vi "IR Opo Main.vi"() -> ()   [LabVIEW 2016] (continued)
          }
        }
        n211 = call "uc480_SubVI_Example_MemoryAllocation.vi"(".NET (Reference)"=w417, "Error In"=w414) -> ("Bits/Pixel 2"=→"Bits/Pixel":i32, "Width"=→"Width":i32, "Serial Number"=→"Serial Number":string, "Height"=→"Height":i32, "Error Out"=w454:errorcluster)  [unwired: 13 in]
      }
      frame "Start live" {
        # "Has acquisition started?"
        # "Start Acquisition"
        n212 = property class="Camera"(reference=w518, error in=w519) -> (error out=w528:errorcluster, "Acquisition"=w527:refnum<k24>)  [unwired: 1 out]
        n213 = invoke class="Acquisition" method="HasStarted"(reference=w527, error in=w528) -> (reference out=w523:refnum<k24>, error out=w522:errorcluster, "HasStarted"=w521:i32, "bValue"=w526:bool)  [unwired: 2 in]
        n214 = control-ref of="Load Parameter"() -> (w511:refnum<vi>)
        n215 = control-ref of="Stop Live"() -> (w509:refnum<vi>)
        n216 = control-ref of="Start Live"() -> (w514:refnum<vi>)
        n217 = property class="Bool"(reference=w514, "Disabled"=u8 2 ("Deaktiviert")) -> (reference out=w503:refnum<vi>, error out=w502:errorcluster)  [unwired: 1 in]
        n218 = property class="Bool"(reference=w511, "Disabled"=u8 2 ("Deaktiviert")) -> (reference out=w505:refnum<vi>, error out=w504:errorcluster)  [unwired: 1 in]
        n219 = invoke class="Acquisition" method="ToString"(reference=w523, error in=w522) -> (error out=w525:errorcluster, "ToString"=w524:string)  [unwired: 1 in, 1 out]
        n220 = property class="Bool"(reference=w509, "Disabled"=u8 0 ("Deaktiviert")) -> (reference out=w507:refnum<vi>, error out=w506:errorcluster)  [unwired: 1 in]
        n221 = call "uc480_Error_Handling.vi"("Error Code"=w521, "Error String"=w524, "Error In"=w525) -> ("Error Out"=w520:errorcluster)  [unwired: 8 in]
        n222 = Close Reference(reference=w507, error in (no error)=w506) -> ()  [unwired: 1 out]
        n223 = Close Reference(reference=w503, error in (no error)=w502) -> ()  [unwired: 1 out]
        n224 = Close Reference(reference=w505, error in (no error)=w504) -> ()  [unwired: 1 out]
        n225 = Get Date/Time In Seconds() -> (seconds since 1Jan1904=w497:timestamp)
        n226 = Format Date/Time String(time format string (%c)="%m/%d/%y - %I:%M %p  ", seconds (now)=w497) -> (date/time string=w496:string)  [unwired: 1 in]
        n227 = Concatenate Strings(w496, "Camera started", "\r") -> (w501:string)
        n228 = invoke on="Log" class="Str" method="Append String"("string"=w501) -> (error out=w494:errorcluster)  [unwired: 3 in, 3 out]
        n229 = property on="Log" class="Str"(error in=w494, "Text.Scroll Position"=u32 500000) -> ()  [unwired: 1 in, 2 out]
        n230 = case shown="False" w526 {
          tunnel: [w531 w541] -> w515
          tunnel: w520 -> [w537 w541]
          tunnel: w518 -> [w536 w540]
          tunnel: [w536 w540] -> w517
          frame False {
            w529 = 1 items=["IS_DONT_WAIT", "IS_WAIT"] ("Wait")
            n231 = property class="Camera"(reference=w536, error in=w537) -> (error out=w538:errorcluster, "Acquisition"=w539:refnum<k24>)  [unwired: 1 out]
            n232 = invoke class="Acquisition" method="Capture"(reference=w539, error in=w538, "param"=w529) -> (reference out=w532:refnum<k24>, error out=w533:errorcluster, "Capture"=w530:i32)  [unwired: 1 in, 1 out]
            n233 = invoke class="Acquisition" method="ToString"(reference=w532, error in=w533) -> (error out=w535:errorcluster, "ToString"=w534:string)  [unwired: 1 in, 1 out]
            n234 = call "uc480_Error_Handling.vi"("Error Code"=w530, "Error String"=w534, "Error In"=w535) -> ("Error Out"=w531:errorcluster)  [unwired: 8 in]
          }
          frame True {
          }
        }
      }
    }
    n235 = call "uc480_SubVI_Example_SyncEventLoop.vi"("Error In"=w55, "use sync"=w57, ".NET (Reference)"=w56) -> ("Error Out"=w53:errorcluster, "Synchronize (ms)"=w54:dbl)  [unwired: 7 in]
    "Error Out" <- w53
    n236 = Wait Until Next ms Multiple(millisecond multiple=w54) -> ()  [unwired: 1 out]
  }
  n237 = flat-sequence "Initialization sequence" {
    tunnel: [w596] -> w20
    tunnel: w20 -> [w658]
    tunnel: [w641] -> w15
    tunnel: [w640] -> w14
    tunnel: [w639] -> w16
    tunnel: [w638] -> w13
    tunnel: [w637] -> w12
    tunnel: w16 -> [w669]
    tunnel: w15 -> [w668]
    tunnel: w14 -> [w667]
    tunnel: [w666] -> w11
    tunnel: w13 -> [w665]
    tunnel: w12 -> [w664]
    tunnel: [w661] -> w10
    tunnel: [w660] -> w6
    tunnel: w11 -> [w689]
    tunnel: [w689] -> w9
    tunnel: w10 -> [w688]
    tunnel: [w687] -> w7
    tunnel: w6 -> [w687]
    tunnel: w9 -> [w699]
    tunnel: [w699] -> w8
    tunnel: w7 -> [w698]
    tunnel: [w708] -> w17
    tunnel: w8 -> [w708]
    tunnel: [w713] -> w18
    tunnel: w17 -> [w713]
    tunnel: [w726] -> w19
    tunnel: w18 -> [w726]
    tunnel: [w728] -> w5
    tunnel: w19 -> [w728]
    tunnel: w5 -> [w732]
    tunnel: [w732] -> w4
    tunnel: w4 -> [w734]
    tunnel: [w734] -> w3
    tunnel: w3 -> [w736]
    tunnel: [w736] -> w2
    tunnel: w2 -> [w738]
    tunnel: [w738] -> w1
    tunnel: w1 -> [w739]
    frame #0 {
      w542 = FALSE ("Visible")
      # "Put name of .ini file here (i.e., opotek_27015_849_847.ini).\nThe .ini file must be in the 'c:\\opotek' directory"
      n238 = control-ref of="This VI"() -> (w570:refnum<vi>)
      n239 = invoke class="VI" method="Default Vals.Reinit All"(reference=w570) -> ()  [unwired: 2 in, 3 out]
      n240 = property on="Axes Manual Control" class="Bool (strict)"("Visible"=w542) -> ()  [unwired: 2 in, 2 out]
      n241 = property on="Home Axes" class="Bool"("Visible"=w542) -> ()  [unwired: 2 in, 2 out]
      n242 = call "File Dialog"("start path"=path "C:/opotek", "pattern (all files)"="*.ini*") -> ("selected path"=w565:path, "cancelled"=w564:bool, "error out"=w563:errorcluster)  [unwired: 10 in, 1 out]
      n243 = case shown="False" w564 {
        tunnel: w563 -> [w579 w581]
        tunnel: [w579 w580] -> w562
        frame False {
          n244 = Get Date/Time In Seconds() -> (seconds since 1Jan1904=w574:timestamp)
          n245 = Format Date/Time String(time format string (%c)="%m/%d/%y -%I:%M %p  ", seconds (now)=w574) -> (date/time string=w573:string)  [unwired: 1 in]
          n246 = Concatenate Strings(w573, "Initializing the OPO laser..." ("Initialiazation"), "\r") -> (w578:string)
          n247 = invoke on="Log" class="Str" method="Append String"("string"=w578) -> (error out=w571:errorcluster)  [unwired: 3 in, 3 out]
          n248 = property on="Log" class="Str"(error in=w571, "Text.Scroll Position"=u32 500000) -> ()  [unwired: 1 in, 2 out]
        }
        frame True {
          n249 = call <vilib>:"Clear Errors.vi"("error in (no error)"=w581) -> ("error out"=w580:errorcluster)  [unwired: 5 in, 1 out]
        }
      }
      n250 = Strip Path(path=w565) -> (name=w568:string)  [unwired: 1 out]
      n251 = dll-call lib="D:/Fabrizio/Labview Projects/IR OPO Controller/Branches/XPS version/OPOTEK.dll" fn="OPOTEK_Init"("INI_File"=w568) -> ("motorCOMPort"=w561:i32, "laserCOMPort"=w560:i32, "error_Code"=→"error_Code":i32)  [unwired: 8 in, 2 out]
      "motorCOMPort" <- w561
      "laserCOMPort" <- w560
      n252 = Number To Decimal String(number=w561) -> (decimal integer string=w559:string)  [unwired: 1 in]
      n253 = Number To Decimal String(number=w560) -> (decimal integer string=w557:string)  [unwired: 1 in]
      n254 = Concatenate Strings("Motor found on port: " ("string"), w559) -> (w555:string)
      n255 = Concatenate Strings("Laser found on port: " ("string"), w557) -> (w554:string)
      n256 = Build Array(w555) -> (w553:string[])
      n257 = Build Array(w554) -> (w552:string[])
      n258 = Build Array(w553, w552) -> (w551:string[][])
      n259 = Get Date/Time In Seconds() -> (seconds since 1Jan1904=w546:timestamp)
      n260 = Format Date/Time String(time format string (%c)="%m/%d/%y -%I:%M %p  ", seconds (now)=w546) -> (date/time string=w545:string)  [unwired: 1 in]
      n261 = Array To Spreadsheet String(array=w551, 3:"%s" ("format string")) -> (spreadsheet string=w548:string)  [unwired: 1 in]
      n262 = Concatenate Strings(w545, w548) -> (w549:string)
      n263 = invoke on="Log" class="Str" method="Append String"("string"=w549) -> (error out=w543:errorcluster)  [unwired: 3 in, 3 out]
      n264 = property on="Log" class="Str"(error in=w543, "Text.Scroll Position"=u32 500000) -> ()  [unwired: 1 in, 2 out]
      n265 = call <vilib>:"Simple Error Handler.vi"("error in (no error)"=w562) -> ()  [unwired: 4 in, 5 out]
    }
    frame #1 {
      w614 = "ROI Processing" ("section")
      w622 = "XPS" ("section")
      n266 = control-ref of="This VI"() -> (w636:refnum<vi>)
      n267 = property class="VI"(reference=w636) -> ("Path"=w634:path)  [unwired: 1 in, 2 out]
      n268 = Strip Path(path=w634) -> (stripped path=w633:path)  [unwired: 1 out]
      n269 = Build Path(base path=w633, name or relative path="General_Configuration.ini") -> (appended path=w624:path)
      n270 = call <vilib>:"Open Config Data.vi"("create file if necessary (T)"=FALSE, "configuration file path"=w624) -> ("error out"=w623:errorcluster, "refnum"=w595:T6)  [unwired: 7 in, 1 out]
      n271 = call-poly <vilib>:"Read Key.vi"("section"="Communication", "default value"="192.168.254.254", "key"="XPSPort", "refnum"=w595) -> ("error out"=w589:errorcluster, "value"=→"XPS_Address":string)  [unwired: 4 in, 2 out]
      n272 = call-poly <vilib>:"Read Key.vi"("section"=w622, "error in (no error)"=w623, "default value"=1.0, "key"="InitialVelocity", "refnum"=w595) -> ("error out"=w588:errorcluster, "value"=→"Velocity":dbl)  [unwired: 3 in, 2 out]
      n273 = call-poly <vilib>:"Read Key.vi"("section"=w622, "default value"=20.0, "key"="Acceleration", "refnum"=w595) -> ("error out"=w587:errorcluster, "value"=→"Acceleration":dbl)  [unwired: 4 in, 2 out]
      n274 = call-poly <vilib>:"Read Key.vi"("section"="Laser" ("key"), "default value"=0, "key"="Wavelenght", "refnum"=w595) -> ("error out"=w586:errorcluster, "value"=→"Default Wavelenght":i32)  [unwired: 4 in, 2 out]
      n275 = Merge Errors(w589, w588, w587, w586) -> (w590:errorcluster)
      n276 = call-poly <vilib>:"Read Key.vi"("section"=w614, "key"="Pixel Size", "refnum"=w595) -> ("error out"=w605:errorcluster, "value"=w594:dbl)  [unwired: 5 in, 2 out]
      n277 = call-poly <vilib>:"Read Key.vi"("section"=w614, "key"="Heigth step divider", "refnum"=w595) -> ("error out"=w604:errorcluster, "value"=w593:i32)  [unwired: 5 in, 2 out]
      n278 = call-poly <vilib>:"Read Key.vi"("section"=w614, "key"="Precision (%)", "refnum"=w595) -> ("error out"=w603:errorcluster, "value"=w591:dbl)  [unwired: 5 in, 2 out]
      n279 = call-poly <vilib>:"Read Key.vi"("section"=w614, "key"="Sampling speed", "refnum"=w595) -> ("error out"=w602:errorcluster, "value"=w592:i32)  [unwired: 5 in, 2 out]
      n280 = call-poly <vilib>:"Read Key.vi"("section"=w614, "key"="Width", "refnum"=w595) -> ("error out"=w601:errorcluster, "value"=w585:i32)  [unwired: 5 in, 2 out]
      n281 = call-poly <vilib>:"Read Key.vi"("section"=w614, "key"="Height", "refnum"=w595) -> ("error out"=w600:errorcluster, "value"=w584:i32)  [unwired: 5 in, 2 out]
      n282 = call-poly <vilib>:"Read Key.vi"("section"=w614, "key"="X offset", "refnum"=w595) -> ("error out"=w599:errorcluster, "value"=w583:i32)  [unwired: 5 in, 2 out]
      n283 = call-poly <vilib>:"Read Key.vi"("section"=w614, "key"="Y offset", "refnum"=w595) -> ("error out"=w598:errorcluster, "value"=w582:i32)  [unwired: 5 in, 2 out]
      n284 = Merge Errors(w605, w604, w603, w602, w601, w600, w599, w598, w590) -> (w597:errorcluster)
      n285 = local write "Height  step \ndivider"(w593) -> ()
      n286 = call <vilib>:"Close Config Data.vi"("error in (no error)"=w597, "refnum"=w595) -> ("error out"=w596:errorcluster)  [unwired: 8 in, 1 out]
      n287 = local write "Speed (µm/s)"(w592) -> ()
      n288 = local write "Precision (%)"(w591) -> ()
      n289 = local write "Pixel size"(w594) -> ()
      n290 = local write "Heigth (µm)"(w584) -> ()
      n291 = local write "Width (µm)"(w585) -> ()
      n292 = local write "Y offset"(w582) -> ()
      n293 = local write "X offset"(w583) -> ()
    }
    frame #2 {
      w642 = "\r"
      n294 = local read "XPS_Address"() -> (w659:string)
      n295 = call <userlib>:"Open TCP-IP.vi"("error in (no error)"=w658, "IP address"=w659) -> ("error out"=w656:errorcluster, "Connection ID"=w657:T7)  [unwired: 4 in, 4 out]
      n296 = call <userlib>:"Objects List Get.vi"("error in (no error)"=w656, "connection ID in"=w657) -> ("error out"=w637:errorcluster, "XPS error out"=w638:errorcluster, "connection ID out"=w639:T7, "Groups"=w655:string[])  [unwired: 4 in, 2 out]
      n297 = Get Date/Time In Seconds() -> (seconds since 1Jan1904=w651:timestamp)
      n298 = Format Date/Time String(time format string (%c)="%m/%d/%y -%I:%M %p  ", seconds (now)=w651) -> (date/time string=w644:string)  [unwired: 1 in]
      n299 = Index Array(array=w655) -> (element=w640:string)  [unwired: 1 in]
      "Axis 1" <- w640
      n300 = Index Array(array=w655, index=1) -> (element=w641:string)
      "Axis 2" <- w641
      n301 = Concatenate Strings(w644, "Axis 1: " ("Initialiazation"), w640, w642) -> (w653:string)
      n302 = Concatenate Strings(w644, "Axis 2: " ("Initialiazation"), w641, w642) -> (w645:string)
      n303 = invoke on="Log" class="Str" method="Append String"("string"=w653) -> (error out=w649:errorcluster)  [unwired: 3 in, 3 out]
      n304 = invoke on="Log" class="Str" method="Append String"("string"=w645) -> (error out=w646:errorcluster)  [unwired: 3 in, 3 out]
      n305 = property on="Log" class="Str"(error in=w649, "Text.Scroll Position"=u32 500000) -> ()  [unwired: 1 in, 2 out]
      n306 = property on="Log" class="Str"(error in=w646, "Text.Scroll Position"=u32 500000) -> ()  [unwired: 1 in, 2 out]
    }
    frame #3 {
      w683 = "Ready"
      n307 = call "Get Stages Status.vi"("error in (no error)"=w664, "XPS error in (no error)"=w665, "Group Name (250 c max)"=w667, "connection ID in"=w669) -> ("error out"=w674:errorcluster, "XPS error out"=w675:errorcluster, "Group Status String"=w671:string, "connection ID out"=w676:T7)  [unwired: 3 in, 1 out]
      n308 = call "Get Stages Status.vi"("error in (no error)"=w674, "XPS error in (no error)"=w675, "Group Name (250 c max)"=w668, "connection ID in"=w676) -> ("error out"=w672:errorcluster, "XPS error out"=w662:errorcluster, "Group Status String"=w670:string, "connection ID out"=w673:T7)  [unwired: 3 in, 1 out]
      n309 = String Subset(string=w671, offset (0)=0, length (rest)=5 ("length (rest)")) -> (substring=w681:string)
      n310 = Bundle(cluster="Axis Initial Parameters", "Velocity (units/seconds)"=5.0) -> (w685:T1)  [unwired: 3 in]
      n311 = call <userlib>:"Close TCP-IP.vi"("error in (no error)"=w672, "connection ID in"=w673) -> ("Error out"=w663:errorcluster)  [unwired: 9 in]
      n312 = local write "Axis Initial Parameters"(w685) -> ()
      n313 = String Subset(string=w670, offset (0)=0, length (rest)=5 ("length (rest)")) -> (substring=w682:string)
      n314 = call <vilib>:"Simple Error Handler.vi"("error in (no error)"=w663) -> ()  [unwired: 4 in, 5 out]
      n315 = call <vilib>:"Simple Error Handler.vi"("error in (no error)"=w662) -> ()  [unwired: 4 in, 5 out]
      n316 = Equal?(x=w681, y=w683) -> (x = y?=w661:bool)
      n317 = Equal?(x=w683, y=w682) -> (x = y?=w660:bool)
      n318 = And(x=w661, y=w660) -> (x .and. y?=w666:bool)
    }
    frame #4 {
      n319 = case shown="True" w688 {
        frame False {
        }
        frame True {
          (unwired) u32 500000 ("Text.Scroll Position")
          n320 = Get Date/Time In Seconds() -> (seconds since 1Jan1904=w694:timestamp)
          n321 = Format Date/Time String(time format string (%c)="%m/%d/%y -%I:%M %p  ", seconds (now)=w694) -> (date/time string=w693:string)  [unwired: 1 in]
          n322 = Concatenate Strings(w693, "Axis 1 ready" ("Initialiazation"), "\r") -> (w691:string)
          n323 = invoke on="Log" class="Str" method="Append String"("string"=w691) -> (error out=w692:errorcluster)  [unwired: 3 in, 3 out]
          n324 = property on="Log" class="Str"(error in=w692, "Text.Scroll Position"=u32 500000) -> ()  [unwired: 1 in, 2 out]
        }
      }
    }
    frame #5 {
      n325 = case shown="True" w698 {
        frame False {
        }
        frame True {
          (unwired) u32 500000 ("Text.Scroll Position")
          n326 = Get Date/Time In Seconds() -> (seconds since 1Jan1904=w704:timestamp)
          n327 = Format Date/Time String(time format string (%c)="%m/%d/%y -%I:%M %p  ", seconds (now)=w704) -> (date/time string=w703:string)  [unwired: 1 in]
          n328 = Concatenate Strings(w703, "Axis 2 ready" ("Initialiazation"), "\r") -> (w701:string)
          n329 = invoke on="Log" class="Str" method="Append String"("string"=w701) -> (error out=w702:errorcluster)  [unwired: 3 in, 3 out]
          n330 = property on="Log" class="Str"(error in=w702, "Text.Scroll Position"=u32 500000) -> ()  [unwired: 1 in, 2 out]
        }
      }
    }
    frame #6 {
      n331 = dll-call lib="D:/Fabrizio/Labview Projects/IR OPO Controller/Branches/XPS version/OPOTEK.dll" fn="OPOTEK_SelectConfiguration"("configuration"=u8 1 ("configuration 2")) -> ("wavelength_Low"=→"Min":dbl, "wavelength_High"=→"Max":dbl, "error_Code"=→"error_Code 2":i32)  [unwired: 8 in, 2 out]
    }
    frame #7 {
      w723 = FALSE ("Visible")
      w719 = u8 1 ("Response to Value Outside Limits:Maximum")
      # "Set defaults"
      n332 = local write "Flash lamp - Q Switch delay (%)"(i16 0 ("Energy")) -> ()
      n333 = local write "Alignment \ndiode"(TRUE ("Alignment diode")) -> ()
      n334 = local write "Repetition \nRate"(enum16{"1", "2", "5", "10", "20"}."20" ("Rep. Rate Divider")) -> ()
      n335 = local read "Max"() -> (w716:dbl)
      n336 = local read "Min"() -> (w717:dbl)
      n337 = call "IR_Alignment_Diode.vi"("AD Action"=enum16{"AD Off", "AD On"}."AD On") -> ()  [unwired: 14 in, 1 out]
      n338 = property on="LAMP" class="Bool (strict)"("BoolText.Text"="LAMP OFF" ("Boolean Text.Text")) -> ()  [unwired: 2 in, 2 out]
      n339 = property on="Laser Operation" class="Bool (strict)"("Blinking"=w723) -> ()  [unwired: 2 in, 2 out]
      n340 = property on="Capture" class="Bool"("Visible"=w723) -> ()  [unwired: 2 in, 2 out]
      n341 = property on="LASER" class="Bool (strict)"("BoolText.Text"="LASER OFF" ("Boolean Text.Text"), "Visible"=FALSE) -> ()  [unwired: 2 in, 2 out]
      n342 = property on="Wavelength" class="DigNum (strict)"("Increment"=1.0 ("Data Entry Limits:Increment"), "Maximum"=w716, "Minimum"=w717, "OutOfRngActMax"=w719, "OutOfRngActMin"=w719) -> ()  [unwired: 2 in, 2 out]
    }
    frame #8 {
      n343 = local read "Default Wavelenght"() -> (w727:i32)
      n344 = local write "Wavelength"(w727) -> ()
      n345 = call "IR_Wavelength_Tuning.vi"("Wavelength (nm)"=w727) -> ()  [unwired: 14 in, 1 out]
    }
    frame #9 {
      w729 = i16 100 ("Energy (0 - 100)")
      n346 = call "IR_Laser_Control.vi"("Action"=T5."Adjust Energy", "Energy (0 - 100)"=w729) -> ()  [unwired: 13 in, 1 out]
      n347 = local write "Flash lamp - Q Switch delay (%)"(w729) -> ()
    }
    frame #10 {
      n348 = local write "Camera Status"("Init camera" ("Camera Status")) -> ()
    }
    frame #11 {
      n349 = Wait (ms)(milliseconds to wait=u32 1000) -> ()  [unwired: 1 out]
    }
    frame #12 {
      n350 = local write "Camera Status"("Start live") -> ()
    }
    frame #13 {
      n351 = Wait (ms)(milliseconds to wait=u32 1000) -> ()  [unwired: 1 out]
    }
    frame #14 {
      n352 = case shown="True" w739 {
        frame False {
          n353 = One Button Dialog(message="Axes not ready") -> ()  [unwired: 1 in, 1 out]
        }
        frame True {
          n354 = Get Date/Time In Seconds() -> (seconds since 1Jan1904=w746:timestamp)
          n355 = property on="Home Axes" class="Bool"("Visible"=TRUE) -> ()  [unwired: 2 in, 2 out]
          n356 = property on="Axes Manual Control" class="Bool (strict)"("Visible"=TRUE) -> ()  [unwired: 2 in, 2 out]
          n357 = Format Date/Time String(time format string (%c)="%m/%d/%y -%I:%M %p  ", seconds (now)=w746) -> (date/time string=w747:string)  [unwired: 1 in]
          n358 = Concatenate Strings(w747, "System ready" ("Initialiazation"), "\r") -> (w749:string)
          n359 = invoke on="Log" class="Str" method="Append String"("string"=w749) -> (error out=w748:errorcluster)  [unwired: 3 in, 3 out]
          n360 = property on="Log" class="Str"(error in=w748, "Text.Scroll Position"=u32 500000) -> ()  [unwired: 1 in, 2 out]
        }
      }
    }
  }
  n361 = while "Laser control & Stages Control" {
    stop <- w761 stop-if-true
    n362 = local read "XPS_Address"() -> (w753:string)
    n363 = local read "Axis 2"() -> (w751:string)
    n364 = local read "Axis 1"() -> (w752:string)
    n365 = event shown="[12] \"Process Image\": Value Change" {
      selector: _ -> [_ _ _ _ _ _ _ _ _ _ _ _ _ _ _ _ _]
      dyn-events: _ -> [_ _ _ _ _ _ _ _ _ _ _ _ _ _ _ _ _]
      timeout: _ -> [_ _ _ _ _ _ _ _ _ _ _ _ _ _ _ _ _]
      tunnel: [_ _ _ _ _ w832 _ _ _ _ _ _ _ _ _ _ _] -> w761
      tunnel: [w765 w772 w791 w814 w821 _ _ _ _ w887 w914 _ w989 "" ("StringOut") w1183 _ w1307] -> w754
      tunnel: w753 -> [_ _ _ _ _ _ _ _ _ _ w917 _ _ w1102 w1182 _ w1294]
      tunnel: w752 -> [_ _ _ _ _ _ _ _ _ _ w916 _ _ w1101 w1181 _ w1293]
      tunnel: w751 -> [_ _ _ _ _ _ _ _ _ _ w915 _ _ w1100 w1180 _ w1292]
      event "Flash lamp - Q Switch delay (%)": Value Change {
        n366 = event-data() -> ()  [unwired: 1 in, 6 out]
        n367 = local read "Flash lamp - Q Switch delay (%)"() -> (w769:i16)
        n368 = call "IR_Laser_Control.vi"("Action"=T5."Adjust Energy", "Energy (0 - 100)"=w769) -> ()  [unwired: 13 in, 1 out]
        n369 = Number To Decimal String(number=w769, width (-)=i16 3) -> (decimal integer string=w767:string)
        n370 = Concatenate Strings("Energy set to: " ("string"), w767) -> (w765:string)
      }
      event "LAMP": Value Change {
        n371 = event-data() -> ()  [unwired: 1 in, 6 out]
        n372 = case shown="True" "LAMP" {
          tunnel: ["Lamp has been switched off" w777] -> w772
          frame False {
            w774 = FALSE ("Visible")
            n373 = property on="LASER" class="Bool (strict)"("Visible"=w774) -> ()  [unwired: 2 in, 2 out]
            n374 = property on="Capture" class="Bool"("Visible"=w774) -> ()  [unwired: 2 in, 2 out]
            n375 = call "IR_Laser_Control.vi"("Action"=T5."Lamp OFF") -> ()  [unwired: 14 in, 1 out]
            n376 = property on="LAMP" class="Bool (strict)"("BoolText.Text"="LAMP OFF" ("Boolean Text.Text")) -> ()  [unwired: 2 in, 2 out]
          }
          frame True {
            n377 = flat-sequence {
              tunnel: ["Lamp has been switched on"] -> w777
              frame #0 {
                n378 = while {
                  i -> [w782]
                  stop <- w785 stop-if-true
                  n379 = Wait Until Next ms Multiple(millisecond multiple=u32 1000) -> ()  [unwired: 1 out]
                  n380 = Equal?(x=10, y=w782) -> (x = y?=w785:bool)
                  n381 = Subtract(x=10, y=w782) -> (x-y=w780:i32)
                  n382 = Number To Decimal String(number=w780) -> (decimal integer string=w781:string)  [unwired: 1 in]
                  n383 = property on="LAMP" class="Bool (strict)"("BoolText.Text"=w781) -> ()  [unwired: 2 in, 2 out]
                }
                n384 = Wait (ms)(milliseconds to wait=u32 10000) -> ()  [unwired: 1 out]
                n385 = call "IR_Laser_Control.vi"("Action"=T5."Lamp ON") -> ()  [unwired: 14 in, 1 out]
              }
              frame #1 {
                w788 = TRUE ("Visible")
                n386 = property on="LASER" class="Bool (strict)"("Visible"=w788) -> ()  [unwired: 2 in, 2 out]
                n387 = property on="Capture" class="Bool"("Visible"=w788) -> ()  [unwired: 2 in, 2 out]
                n388 = property on="LAMP" class="Bool (strict)"("BoolText.Text"="LAMP ON" ("Boolean Text.Text")) -> ()  [unwired: 2 in, 2 out]
              }
            }
          }
        }
      }
      event "LASER": Value Change {
        n389 = event-data() -> ()  [unwired: 1 in, 6 out]
        n390 = case shown="True" "LASER" {
          tunnel: [w796 w802] -> w792
          tunnel: ["Q-Switch has switched off" w801] -> w791
          frame False {
            w796 = FALSE ("Boolean")
            n391 = local read "Alignment \ndiode"() -> (w793:bool)
            n392 = property on="Capture" class="Bool"("Visible"=TRUE) -> ()  [unwired: 2 in, 2 out]
            n393 = case shown="False" w793 {
              frame False {
                n394 = call "IR_Alignment_Diode.vi"("AD Action"=enum16{"AD Off", "AD On"}."AD Off") -> ()  [unwired: 14 in, 1 out]
              }
              frame True {
                n395 = call "IR_Alignment_Diode.vi"("AD Action"=enum16{"AD Off", "AD On"}."AD On") -> ()  [unwired: 14 in, 1 out]
              }
            }
            n396 = call "IR_Laser_Control.vi"("Action"=T5."Q-switch OFF") -> ()  [unwired: 14 in, 1 out]
            n397 = property on="LASER" class="Bool (strict)"("BoolText.Text"="LASER OFF" ("Boolean Text.Text"), "Value"=w796) -> ()  [unwired: 2 in, 2 out]
            n398 = property on="Laser Operation" class="Bool (strict)"("Blinking"=w796) -> ()  [unwired: 2 in, 2 out]
          }
          frame True {
            n399 = property on="LAMP" class="Bool (strict)"() -> ("BoolText.Text"=w805:string)  [unwired: 2 in, 2 out]
            n400 = Equal?(x=w805, y="LAMP ON") -> (x = y?=w803:bool)
            n401 = case shown="True" w803 {
              tunnel: [FALSE ("Boolean") w811] -> w802
              tunnel: ["Q-Switch has switched off" "Q-Switch has switched on"] -> w801
              frame False {
              }
              frame True {
                w811 = TRUE ("Boolean")
                n402 = property on="Capture" class="Bool"("Visible"=FALSE) -> ()  [unwired: 2 in, 2 out]
                n403 = property on="LASER" class="Bool (strict)"("BoolText.Text"="LASER ON" ("Boolean Text.Text")) -> ()  [unwired: 2 in, 2 out]
                n404 = call "IR_Alignment_Diode.vi"("AD Action"=enum16{"AD Off", "AD On"}."AD Off") -> ()  [unwired: 14 in, 1 out]
                n405 = property on="Laser Operation" class="Bool (strict)"("Blinking"=w811) -> ()  [unwired: 2 in, 2 out]
                n406 = call "IR_Laser_Control.vi"("Action"=T5."Q-switch ON") -> ()  [unwired: 14 in, 1 out]
              }
            }
          }
        }
        "Laser Operation" <- w792
      }
      event "Repetition \nRate": Value Change {
        n407 = event-data() -> ()  [unwired: 1 in, 6 out]
        n408 = local read "Repetition \nRate"() -> (w815:enum16{"1", "2", "5", "10", "20"})
        n409 = call "IR_Laser_Control.vi"("Action"=T5."Change Rep. Rate", "Rep. Rate Divider"=w815) -> ()  [unwired: 13 in, 1 out]
        n410 = Number To Decimal String(number=w815, width (-)=i16 3) -> (decimal integer string=w817:string)
        n411 = Concatenate Strings("Repetition rate set to: " ("string"), w817) -> (w814:string)
      }
      event "Tune": Value Change {
        n412 = event-data() -> ()  [unwired: 1 in, 6 out]
        n413 = case shown="True" "Tune" {
          tunnel: [_ w822] -> w821
          frame False {
          }
          frame True {
            n414 = property on="LASER" class="Bool (strict)"() -> ("BoolText.Text"=w829:string)  [unwired: 2 in, 2 out]
            n415 = Equal?(x=w829, y="LASER ON") -> (x = y?=w827:bool)
            n416 = case shown="False" w827 {
              tunnel: [w830 w831] -> w823
              frame False {
                n417 = local read "Wavelength"() -> (w830:dbl)
                n418 = call "IR_Wavelength_Tuning.vi"("Wavelength (nm)"=w830) -> ()  [unwired: 14 in, 1 out]
              }
              frame True {
                n419 = local read "Wavelength"() -> (w831:dbl)
              }
            }
            n420 = Number To Decimal String(number=w823, width (-)=i16 3) -> (decimal integer string=w825:string)
            n421 = Concatenate Strings("Wavelength set to: " ("string"), w825) -> (w822:string)
          }
        }
      }
      event "EXIT": Value Change {
        n422 = event-data() -> ()  [unwired: 1 in, 6 out]
        n423 = flat-sequence {
          tunnel: ["EXIT"] -> w832
          frame #0 {
            n424 = call "IR_Laser_Control.vi"("Action"=T5."Lamp OFF") -> ()  [unwired: 14 in, 1 out]
          }
          frame #1 {
            n425 = Wait (ms)(milliseconds to wait=u32 1000) -> ()  [unwired: 1 out]
          }
          frame #2 {
            n426 = dll-call lib="D:/Fabrizio/Labview Projects/IR OPO Controller/Branches/XPS version/OPOTEK.dll" fn="OPOTEK_Close"() -> ("error_Code"=→"error_Code 3":i32)  [unwired: 5 in, 2 out]
          }
          frame #3 {
            n427 = Wait (ms)(milliseconds to wait=u32 1000) -> ()  [unwired: 1 out]
          }
          frame #4 {
            n428 = local write "Camera Status"("Exit camera") -> ()
          }
          frame #5 {
            n429 = Wait (ms)(milliseconds to wait=u32 1000) -> ()  [unwired: 1 out]
          }
          frame #6 {
            n430 = control-ref of="This VI"() -> (w842:refnum<vi>)
            n431 = property class="VI"(reference=w842) -> ("Path"=w843:path)  [unwired: 1 in, 2 out]
            n432 = control-ref of="This Application"() -> (w858:refnum<vi>)
            n433 = Strip Path(path=w843) -> (stripped path=w852:path)  [unwired: 1 out]
            n434 = property class="App"(reference=w858) -> ("App.Kind"=w857:T10)  [unwired: 1 in, 2 out]
            n435 = Build Path(base path=w852, name or relative path="Logs") -> (appended path=w850:path)
            n436 = case shown="\"Run Time System\"" w857 {
              frame "Development System", Default {
              }
              frame "Run Time System" {
                n437 = control-ref of="This VI"() -> (w867:refnum<vi>)
                n438 = invoke class="VI" method="FP.Close"(reference=w867) -> ()  [unwired: 2 in, 3 out]
                n439 = Quit LabVIEW() -> ()  [unwired: 1 in]
              }
            }
            n440 = call <vilib>:"Check if File or Folder Exists.vi"("path"=w850) -> ("file or folder exists?"=w851:bool, "dup path"=w853:path)  [unwired: 8 in, 1 out]
            n441 = case shown="True" w851 {
              tunnel: w853 -> [w860 w861]
              tunnel: [w859 w861] -> w856
              frame False {
                n442 = Create Folder(path (use dialog)=w860) -> (created path=w859:path)  [unwired: 2 in, 2 out]
              }
              frame True {
              }
            }
            n443 = Get Date/Time In Seconds() -> (seconds since 1Jan1904=w847:timestamp)
            n444 = Format Date/Time String(time format string (%c)="%d%m%y %I-%M %p ", seconds (now)=w847) -> (date/time string=w845:string)  [unwired: 1 in]
            n445 = Concatenate Strings(w845, "Log File.txt") -> (w855:string)
            n446 = Build Path(base path=w856, name or relative path=w855) -> (appended path=w854:path)
            n447 = Open/Create/Replace File(file path (use dialog)=w854, operation (0:open)=T8."replace or create") -> (refnum out=w841:refnum<file>, cancelled=w839:bool, error out=w840:errorcluster)  [unwired: 4 in]
            n448 = case shown="False" w839 {
              tunnel: w841 -> [w866 _]
              tunnel: w840 -> [w864 _]
              frame False {
                n449 = local read "Log"() -> (w865:string)
                n450 = Write to Text File(file (use dialog)=w866, text=w865, error in=w864) -> (refnum out=w863:refnum<file>, error out=w862:errorcluster)  [unwired: 2 out]
                n451 = Close File(refnum=w863, error in=w862) -> ()  [unwired: 2 out]
              }
              frame True {
              }
            }
          }
          frame #7 {
          }
        }
      }
      event "Processing time unit", "Processi time (sec)": Value Change {
        n452 = event-data() -> ()  [unwired: 1 in, 6 out]
        n453 = local read "Processing time unit"() -> (w871:string)
        n454 = Equal?(x=w871, y="min") -> (x = y?=w869:bool)
        n455 = case shown="False" w869 {
          frame False {
            n456 = local read "Processi time (sec)"() -> (w872:i32)
            n457 = local write "Process time"(w872) -> ()
          }
          frame True {
            n458 = local read "Processi time (sec)"() -> (w874:i32)
            n459 = Quotient & Remainder(x=w874, y=60) -> (floor(x/y)=w873:i32)  [unwired: 1 out]
            n460 = local write "Process time"(w873) -> ()
          }
        }
      }
      event "Overlay MSI Image": Value Change {
        n461 = event-data() -> ()  [unwired: 1 in, 6 out]
        n462 = case shown="True" "Overlay MSI Image" {
          frame False {
          }
          frame True {
            n463 = vi-ref "MSI_Image_overlap.vi"() -> (w882:refnum<vi>)
            n464 = invoke class="VI" method="FP.Open"(reference=w882, "Activate"=TRUE ("Activate?"), "State"=T9."Standard") -> (reference out=w879:refnum<vi>)  [unwired: 2 in, 4 out]
            n465 = invoke class="VI" method="Run VI"(reference=w879, "Wait until done"=FALSE ("Wait Until Done"), "Auto Dispose Ref"=TRUE ("Auto Dispose Reference")) -> ()  [unwired: 2 in, 5 out]
          }
        }
      }
      event "Alignment \ndiode": Value Change {
        n466 = event-data() -> ()  [unwired: 1 in, 6 out]
        n467 = case shown="False" "Alignment \ndiode" {
          frame False {
            n468 = call "IR_Alignment_Diode.vi"("AD Action"=enum16{"AD Off", "AD On"}."AD Off") -> ()  [unwired: 14 in, 1 out]
          }
          frame True {
            n469 = call "IR_Alignment_Diode.vi"("AD Action"=enum16{"AD Off", "AD On"}."AD On") -> ()  [unwired: 14 in, 1 out]
          }
        }
      }
      event "Open \nManual": Value Change {
        n470 = event-data() -> ()  [unwired: 1 in, 6 out]
        n471 = case shown="True" "Open \nManual" {
          tunnel: [_ "Opening Manual" ("StringOut")] -> w887
          frame False {
          }
          frame True {
            w896 = FALSE  # wait until completion? (T)
            n472 = control-ref of="This VI"() -> (w900:refnum<vi>)
            n473 = property class="VI"(reference=w900) -> ("Path"=w899:path)  [unwired: 1 in, 2 out]
            n474 = Strip Path(path=w899) -> (stripped path=w898:path)  [unwired: 1 out]
            n475 = Build Path(base path=w898, name or relative path="LAST_Software_Manual.PDF") -> (appended path=w890:path)
            n476 = Path To String(path=w890) -> (string=w893:string)
            n477 = Concatenate Strings("cmd  /c \"", w893, "\"" ("string")) -> (w888:string)
            n478 = call <vilib>:"System Exec.vi"("run minimized? (F)"=TRUE, "wait until completion? (T)"=w896, "error in (no error)"="error in (no error)", "command line"=w888) -> ("error out"=→"error out":errorcluster)  [unwired: 4 in, 3 out]
          }
        }
      }
      event "Stages status": Value Change {
        w908 = "Ready"
        n479 = event-data() -> ()  [unwired: 1 in, 6 out]
        n480 = case shown="True" "Stages status" {
          tunnel: w917 -> [_ w930]
          tunnel: w916 -> [_ w929]
          tunnel: w915 -> [_ w928]
          tunnel: [w921 w927] -> w914
          tunnel: [w921 w925] -> w904
          tunnel: [w921 w926] -> w903
          frame False {
            w921 = ""
          }
          frame True {
            n481 = call <userlib>:"Open TCP-IP.vi"("IP address"=w930) -> ("error out"=w924:errorcluster, "Connection ID"=w931:T7)  [unwired: 8 in, 1 out]
            n482 = call <vilib>:"Simple Error Handler.vi"("error in (no error)"=w924) -> ("error?"=w922:bool, "error out"=w923:errorcluster)  [unwired: 4 in, 3 out]
            n483 = case shown="True" w922 {
              tunnel: w931 -> [w952 _]
              tunnel: w923 -> [w951 _]
              tunnel: w929 -> [w944 _]
              tunnel: w928 -> [w943 _]
              tunnel: [w942 w953] -> w927
              tunnel: [w939 w953] -> w926
              tunnel: [w935 w953] -> w925
              frame False {
                n484 = call "Get Stages Status.vi"("error in (no error)"=w951, "Group Name (250 c max)"=w944, "connection ID in"=w952) -> ("error out"=w948:errorcluster, "XPS error out"=w947:errorcluster, "Group Status String"=w939:string, "connection ID out"=w950:T7)  [unwired: 4 in, 1 out]
                n485 = call "Get Stages Status.vi"("error in (no error)"=w948, "XPS error in (no error)"=w947, "Group Name (250 c max)"=w943, "connection ID in"=w950) -> ("error out"=w945:errorcluster, "XPS error out"=w941:errorcluster, "Group Status String"=w935:string, "connection ID out"=w946:T7)  [unwired: 3 in, 1 out]
                n486 = call <vilib>:"Simple Error Handler.vi"("error source (\" \")"="Stage status" ("error source (\" \")"), "error in (no error)"=w941) -> ()  [unwired: 3 in, 5 out]
                n487 = Concatenate Strings("Axis 1 " ("string"), w939) -> (w938:string)
                n488 = call <userlib>:"Close TCP-IP.vi"("error in (no error)"=w945, "connection ID in"=w946) -> ("Error out"=w940:errorcluster)  [unwired: 9 in]
                n489 = call <vilib>:"Simple Error Handler.vi"("error source (\" \")"="TCP close Stage status" ("error source (\" \")"), "error in (no error)"=w940) -> ()  [unwired: 3 in, 5 out]
                n490 = Concatenate Strings("Axis 2 " ("string"), w935) -> (w936:string)
                n491 = Concatenate Strings(w938, " - " ("string"), w936) -> (w942:string)
              }
              frame True {
                w953 = ""
              }
            }
          }
        }
        n492 = String Subset(string=w903, offset (0)=0, length (rest)=5 ("length (rest)")) -> (substring=w907:string)
        n493 = String Subset(string=w904, offset (0)=0, length (rest)=5 ("length (rest)")) -> (substring=w909:string)
        n494 = Equal?(x=w908, y=w907) -> (x = y?=w905:bool)
        n495 = Equal?(x=w909, y=w908) -> (x = y?=w906:bool)
        n496 = And(x=w906, y=w905) -> (x .and. y?=w902:bool)
        n497 = case shown="True" w902 {
          frame False {
          }
          frame True {
            n498 = property on="Axes Manual Control" class="Bool (strict)"("Visible"=TRUE) -> ()  [unwired: 2 in, 2 out]
            n499 = property on="Home Axes" class="Bool"("Visible"=TRUE) -> ()  [unwired: 2 in, 2 out]
          }
        }
      }
      event "Save configuration": Value Change {
        n500 = event-data() -> ()  [unwired: 1 in, 6 out]
        n501 = case shown="True" "Save configuration" {
          frame False {
          }
          frame True {
            w981 = "ROI Processing" ("section")
            n502 = control-ref of="This VI"() -> (w987:refnum<vi>)
            n503 = property class="VI"(reference=w987) -> ("Path"=w986:path)  [unwired: 1 in, 2 out]
            n504 = Strip Path(path=w986) -> (stripped path=w985:path)  [unwired: 1 out]
            n505 = Build Path(base path=w985, name or relative path="General_Configuration.ini") -> (appended path=w983:path)
            n506 = local read "Heigth (µm)"() -> (w967:i32)
            n507 = local read "Width (µm)"() -> (w968:i32)
            n508 = local read "Pixel size"() -> (w979:dbl)
            n509 = local read "X offset"() -> (w966:i32)
            n510 = local read "Y offset"() -> (w965:i32)
            n511 = local read "Height  step \ndivider"() -> (w978:i32)
            n512 = call <vilib>:"Open Config Data.vi"("create file if necessary (T)"=FALSE, "configuration file path"=w983) -> ("refnum"=w955:T6)  [unwired: 7 in, 2 out]
            n513 = local read "Speed (µm/s)"() -> (w969:i32)
            n514 = local read "Precision (%)"() -> (w970:dbl)
            n515 = call-poly <vilib>:"Write Key.vi"("section"=w981, "value"=w979, "key"="Pixel Size", "refnum"=w955) -> ("error out"=w964:errorcluster)  [unwired: 5 in, 2 out]
            n516 = call-poly <vilib>:"Write Key.vi"("section"=w981, "value"=w978, "key"="Heigth step divider", "refnum"=w955) -> ("error out"=w963:errorcluster)  [unwired: 5 in, 2 out]
            n517 = call-poly <vilib>:"Write Key.vi"("section"=w981, "value"=w970, "key"="Precision (%)", "refnum"=w955) -> ("error out"=w962:errorcluster)  [unwired: 5 in, 2 out]
            n518 = call-poly <vilib>:"Write Key.vi"("section"=w981, "value"=w969, "key"="Sampling speed", "refnum"=w955) -> ("error out"=w961:errorcluster)  [unwired: 5 in, 2 out]
            n519 = call-poly <vilib>:"Write Key.vi"("section"=w981, "value"=w968, "key"="Width", "refnum"=w955) -> ("error out"=w960:errorcluster)  [unwired: 5 in, 2 out]
            n520 = call-poly <vilib>:"Write Key.vi"("section"=w981, "value"=w967, "key"="Height", "refnum"=w955) -> ("error out"=w959:errorcluster)  [unwired: 5 in, 2 out]
            n521 = call-poly <vilib>:"Write Key.vi"("section"=w981, "value"=w966, "key"="X offset", "refnum"=w955) -> ("error out"=w958:errorcluster)  [unwired: 5 in, 2 out]
            n522 = call-poly <vilib>:"Write Key.vi"("section"=w981, "value"=w965, "key"="Y offset", "refnum"=w955) -> ("error out"=w957:errorcluster)  [unwired: 5 in, 2 out]
            n523 = Merge Errors(w964, w963, w962, w961, w960, w959, w958, w957) -> (w956:errorcluster)
            n524 = call <vilib>:"Close Config Data.vi"("error in (no error)"=w956, "refnum"=w955) -> ()  [unwired: 8 in, 2 out]
          }
        }
      }
      event "Process Image": Value Change {
        n525 = event-data() -> ()  [unwired: 1 in, 6 out]
        n526 = case shown="True" "Process Image" {
          tunnel: ["" "Processing done"] -> w989
          frame False {
          }
          frame True {
            w1016 = 0.5  # Delay after laser on/off
            w1028 = 2.0 ("y")
            w1065 = T11 0 items=["Grayscale (U8)", "Grayscale (I16)", "Grayscale (SGL)", "Complex (CSG)", "RGB (U32)", "HSL (U32)", "RGB (U64)", "Grayscale (U16)"] ("Image Type")
            w1068 = i16 4 ("precision (6)")
            w1060 = 1000 ("y")
            n527 = local read "Source"() -> (w1067:T2)
            n528 = property on="Source" class="ImageControl"() -> ("ROI"=w1071:T12)  [unwired: 2 in, 2 out]
            n529 = call "IMAQ Cast Image"("Image Type"=w1065, "Image Src"=w1067) -> ("error out"=w996:errorcluster, "Image Dst Out"=w1066:T2)  [unwired: 8 in]
            n530 = Unbundle By Name(w1071) -> ("Global Rectangle"=w1001:i32[])
            n531 = call "IMAQ ROIToMask 2"("error in (no error)"=w996, "ROI Descriptor"=w1071, "Image"=w1066) -> ("error out"=w997:errorcluster, "Image Out"=w1073:T2)  [unwired: 6 in, 1 out]
            n532 = call "IMAQ ImageToArray"("error in (no error)"=w997, "Image"=w1073) -> ("error out"=w995:errorcluster, "Image Pixels (U8)"=w1050:u8[][])  [unwired: 2 in, 3 out]
            n533 = Array To Cluster(array=w1001) -> (cluster=w1000:T13)
            n534 = local read "X offset"() -> (w1063:i32)
            n535 = local read "Y offset"() -> (w1064:i32)
            n536 = call <vilib>:"Simple Error Handler.vi"("error in (no error)"=w995) -> ()  [unwired: 4 in, 5 out]
            n537 = Unbundle(w1000) -> ("Global Rectangle[0]"=w999:i32, "Global Rectangle[1]"=w998:i32)
            n538 = Empty Array?(array=w1050) -> (empty?=w1051:bool)
            n539 = Subtract(x=w999, y=w1063) -> (x-y=w1070:i32)
            n540 = Subtract(x=w998, y=w1064) -> (x-y=w1069:i32)
            n541 = case shown="False" w1051 {
              tunnel: [w1091 u8[][] [[1]] ("Image Pixels (U8)")] -> w1049
              tunnel: w1050 -> [w1091 _]